vi "UHR-Fleezers Control (host) - 12.7b.vi"() -> ()   [LabVIEW 2012] (continued)
  T23 = typedef "XDNodeRunTimeDep.lvlib/timing_clust.ctl" = cluster{"Expected End [f-1]":u64, "Actual End [f-1]":u64, "Finished Late? [f-1]":bool, "Expected End [i-1]":u64, "Actual End [i-1]":u64, "Finished Late? [i-1]":bool, "Expected Start [i]":u64, "Actual Start [i]":u64, "Expected Start [f]":u64, "Actual Start [f]":u64, "Source Name":string, "Structure Name":string, "Period":i64, "Deadline":i64, "Offset":i64, "Start":i64, "Priority":i32, "Timeout":i32, "Mode":T24, "Wakeup Reason":T25, "Error":errorcluster, "Source Type":string, "Secondary Source Type":string, "Global End Time":u64, "Global Start Time":u64, "Frame Duration":u64, "Iteration Duration":u64, "Assigned CPU":i32, "I/O Scan Engine Mode":u32}
  T24 = typedef "XDNodeRunTimeDep.lvlib/nitl_modes.ctl" = enum32{"No Change", "Process missed periods, maintain original phase", "Discard missed periods, maintain original phase", "Process missed periods, ignore original phase", "Discard missed periods, ignore original phase"}
  T25 = typedef "XDNodeRunTimeDep.lvlib/wakeup.ctl" = enum32{"Normal", "Aborted", "Asynchronous wakeup", "Timing source error", "Timed loop error", "Timeout"}
  T26 = enum32{"Status", "Sample Stage", "Syringe Pump", "Trap Control (RF)", "APD Counting", "Fluorescence Laser Control", "Trap AI", "Video", "FPGA"}
  T27 = enum32{"Status", "Sample Stage", "Syringe Pump", "Trap Control (RF)", "APD Counting", "Fluorescence Laser Control", "Trap AI", "Video", "FPGA", "Misc. Configuration"}
  T28 = enum16{"big-endian, network order", "native, host order", "little-endian"}
  T29 = enum16{"open", "replace", "create", "open or create", "replace or create", "replace or create with confirmation"}
  T30 = cluster{"Scan Range AOD (nm) 2":dbl, "Step Size AOD (nm) 2":dbl, "Scan Speed AOD (nm/s) 2":dbl, "Number of scans (AOD) 2":u16, "Label":string}
  T31 = cluster{"[0]":dbl, "[1]":dbl, "[2]":dbl, "[3]":dbl, "[4]":dbl, "[5]":dbl}
  T32 = cluster{"Diameter (mm)":dbl, "Units":dbl, "Volume":dbl, "Rate":dbl}
  T33 = cluster{"Left":i32, "Top":i32, "Width":u32, "Height":u32}
  T34 = cluster{cluster{"Left":i32, "Top":i32, "Width":u32, "Height":u32}}[]
  T35 = enum32{"Normal Display", "Dual Display (APD)", "FFT", "High Res Display"}
  T36 = cluster{"Origin Pixel":cluster{"X":sgl, "Y":sgl}, "Angle Relative to Horizontal (deg)":sgl, "Axis Reference":u32}
  T37 = typedef "Simple Grid Descriptor" = cluster{"X Step":sgl, "Y Step":sgl, "Unit":T38}
  T38 = typedef "Image Unit" = enum32{"Undefined", "Angström", "Micrometer", "Millimeter", "Centimeter", "Meter", "Kilometer", "Microinch", "Inch", "Feet", "Nautical miles", "Standard miles", "Steps"}
  T39 = cluster{"averaging mode":u16, "weighting mode":u16, "number of averages":u32}
  T40 = cluster{"dB On (F)":bool, "unwrap phase (F)":bool, "convert to degree (F)":bool}
  T41 = cluster{string, string, string, string, string, string, string, string}
  T42 = cluster{string, string, string, string, string, string, string, string, string, string, string, string}
  T43 = cluster{string, string, string, string, string, string, string, string, string, string, string, string, string}
  T44 = cluster{string, string, string, string, string, string, string, string, string, string, string, string, string, string}
  T45 = cluster{"BD 1 Frequency 1 (MHz)":dbl, "BD 1 Frequency 2 (MHz)":dbl}
  T46 = cluster{"f0":dbl, "df":dbl, "magnitude":dbl[]}[][]
  T47 = cluster{"Comment (data description)":string, "Channel 1 Buffer":string, "Channel 2 Buffer":string, "Channel 3 Buffer":string, "Title":string, "DNA Construct":string, "Bead diameter":dbl, "Name":string}
  T48 = enum32{"setting", "request", "request control", "info", "statistics", "system settings", "I/O sub system", "HRT control", "camera descriptions", "device specific data", "event sub system settings", "event sub system results", "image memory manager"}
  T49 = typedef "AviRefnum.ctl" = refnum<k1>
  T50 = typedef "imagedata.ctl" = cluster{"image type":i32, "image depth":i32, "image":u8[], "mask":u8[], "colors":u32[], "Rectangle":cluster{"left":i16, "top":i16, "right":i16, "bottom":i16}}
diagram:
  w13 = u16 10 items=["1.0"=10, "1.5"=15, "2.0"=20] ("stop bits (10: 1 bit)")
  w80 = u16 20 items=["1.0"=10, "1.5"=15, "2.0"=20] ("stop bits (10: 1 bit)")
  w83 = u16 20 items=["1.0"=10, "1.5"=15, "2.0"=20] ("stop bits (10: 1 bit)")
  w109 = u16 20 items=["1.0"=10, "1.5"=15, "2.0"=20] ("stop bits (10: 1 bit)")
  w19 = T18 2 items=["Grayscale (U8)", "Grayscale (I16)", "Grayscale (SGL)", "Complex (CSG)", "RGB (U32)", "HSL (U32)", "RGB (U64)", "Grayscale (U16)"] ("Image Type")
  w239 = 10.0 ("y")
  w238 = 32767.0 ("y")
  w254 = 6.0  # clock mult.
  w255 = 49152000.0  # TCXO frequ.
  # "Trap X limits"
  # "What are these?"
  # "I don't think you need to do this.\nEverytime you want to adjust phase you always set this anyway.\nSince we removed the separate +/- controls.\n\nHaven't added for added fl lasers.  Should remove this code."
  # "Bottom 1 Harvard"
  # "Top 3 Harvard"
  # "Center Harvard"
  # "Bottom 1 Harvard"
  # "Top 3 Harvard"
  # "Center Harvard"
  n1 = Build Array("DIO count 1 (ticks)", "DIO count 2 (ticks)", "DIO count 3 (ticks)") -> (w160:u16[])
  n2 = xnode "Open FPGA VI Reference"("resource name"=T19 "750kHzDAQ") -> ("FPGA VI Reference Out"=w263:T20, "error out"=w262:errorcluster)  [unwired: 1 in]
  n3 = local read "AO1"() -> (w233:dbl)
  n4 = local read "AO2"() -> (w232:dbl)
  n5 = local read "Scan Increment (MHz)"() -> (w250:dbl)
  n6 = local read "Continuous MCL Scanning"() -> (w220:bool)
  n7 = local read "Fast Scan Dir"() -> (w219:bool)
  n8 = xnode "Invoke Method"("FPGA VI Reference In"=w263, "error in"=w262) -> ("FPGA VI Reference Out"=w23:T20, "error out"=w179:errorcluster)
  n9 = local read "Number of scans (MCL)"() -> (w221:u64)
  n10 = Multiply(x=w233, y=w238) -> (x*y=w235:dbl)
  n11 = Multiply(x=w232, y=w238) -> (x*y=w237:dbl)
  n12 = Divide(x=w235, y=w239) -> (x/y=w234:dbl)
  n13 = Divide(x=w237, y=w239) -> (x/y=w236:dbl)
  n14 = To Word Integer(number=w234) -> (16bit integer=w231:i16)
  n15 = To Word Integer(number=w236) -> (16bit integer=w230:i16)
  n16 = Not(x=w219) -> (.not. x?=w214:bool)
  n17 = local read "Cycles/step (MCL)"() -> (w222:u64)
  n18 = Multiply(x=w250, y=1000.0) -> (x*y=w257:dbl)
  n19 = local read "Scan steps (MCL)"() -> (w223:u64)
  n20 = local read "Desired Scan Incr (V)"() -> (w225:dbl)
  n21 = Scale By Power Of 2(n=48, x=w257) -> (x*2^n=w258:dbl)
  n22 = Unbundle By Name(cluster{"output high":i16, "output low":i16} {"output high"=3000, "output low"=0} ("FB output range 1")) -> ("output high"=w61:i16, "output low"=w60:i16)
  n23 = Multiply(x=w255, y=w254) -> (x*y=w253:dbl)
  n24 = Divide(x=w258, y=w253) -> (x/y=w252:dbl)
  n25 = local read "Setpoints (V)"() -> (w269:cluster{"Set 1":dbl, "Set 2":dbl})
  n26 = To Quad Integer(1:w252) -> (0:w249:i64)
  n27 = Divide(x=40000000.0, y="AI Count (ticks)") -> (x/y=w210:dbl)
  n28 = Multiply(x=w225, y=32767.0) -> (x*y=w227:dbl)
  n29 = local read "Trap Intensity PID Gains"() -> (w264:T9)
  n30 = local read "Next trap write delay (ticks)"() -> (w5:u8)
  n31 = local read "XY phase ext loop method"() -> (w4:bool)
  n32 = local read "Amp switch delay 2"() -> (w3:u8)
  n33 = local read "BD 2 Delay (Ticks) 2"() -> (w2:u8)
  n34 = local read "BD 1 Delay (ticks) 2"() -> (w1:u8)
  n35 = local write "Trap Pos FIFO Timeout"(u16 0 ("Trap Pos FIFO Timeout")) -> ()
  n36 = local read "Number Interlace Sets"() -> (w153:u8)
  n37 = Split 1D Array(array=w160, index=w153) -> (first subarray=w162:u16[])  [unwired: 1 out]
  n38 = Add Array Elements(numeric array=w162) -> (sum=w161:u16)
  n39 = local read "# Samples/channel"() -> (w242:u32)
  n40 = local read "Number of F/B Scans (AOD)"() -> (w243:u16)
  n41 = local read "Not-Interlacing Set"() -> (w152:enum32{"Set 1", "Set 2", "Set 3"})
  n42 = To Unsigned Byte Integer(number=w152) -> (unsigned 8bit integer=w158:u8)
  n43 = Index Array(array=w160, index=w158) -> (element=w159:u16)
  n44 = local read "Feedback On/Off"() -> (w272:cluster{"Set 1":bool, "Set 2":bool})
  n45 = local read "BD 2 Delay (Ticks)"() -> (w6:u8)
  n46 = local read "BD 1 Delay (ticks)"() -> (w7:u8)
  n47 = local read "Scan steps (AOD)"() -> (w248:u64)
  n48 = local read "All FB On/Off"() -> (w273:bool)
  n49 = local read "Cycles/step (AOD)"() -> (w247:u64)
  n50 = local write "AI rate (Hz)"(w210) -> ()
  n51 = Divide(x=w227, y=10.0) -> (x/y=w226:dbl)
  n52 = Multiply(x=w248, y=w247) -> (x*y=w246:u64)
  n53 = Unbundle By Name(w264) -> ("proportional gain (Kc)"=w65:i16, "integral gain (Kc*Ts/Ti)"=w64:i16, "derivative gain (Kc*Td/Ts)"=w63:i16)
  n54 = property on="AI Count (ticks)" class="DigNum (strict)"("Val(Sgnl)"="AI Count (ticks)") -> ()  [unwired: 2 in, 2 out]
  n55 = Multiply(x=3276.7, y=w269) -> (x*y=w268:cluster{"Set 1":dbl, "Set 2":dbl})
  n56 = To Word Integer(number=w226) -> (16bit integer=w224:i16)
  n57 = Multiply(x=w246, y=u64 2) -> (x*y=w244:u64)
  n58 = Divide(x=w210, y="FPGA Ave.") -> (x/y=w211:dbl)
  n59 = To Word Integer(number=w268) -> (16bit integer=w267:cluster{"Set 1":i16, "Set 2":i16})
  n60 = Multiply(x=w244, y=w243) -> (x*y=w241:u64)
  n61 = local read "Sets to FIFO (Traps)"() -> (w69:T15)
  n62 = local write "Ave. Rate (Hz)"(w211) -> ()
  n63 = Divide(x=w241, y=w242) -> (x/y=w240:dbl)
  n64 = Unbundle By Name(w267) -> ("Set 1"=w266:i16, "Set 2"=w265:i16)
  n65 = local read "2D or 1D Scan"() -> (w171:bool)
  n66 = local write "Data points/scans"(w241) -> ()
  n67 = local read "Scan BD"() -> (w259:bool)
  n68 = And(x=w272, y=w273) -> (x .and. y?=w271:cluster{"Set 1":bool, "Set 2":bool})
  n69 = local write "Data points/scan (f/b)"(w244) -> ()
  n70 = Reciprocal(x=w211) -> (1/x=w212:dbl)
  n71 = local read "N Acq Sets (Traps + Fl.)"() -> (w203:i16)
  n72 = local write "N sets should be saved"(w240) -> ()
  n73 = Unbundle By Name(w271) -> ("Set 1"=w275:bool, "Set 2"=w274:bool)
  n74 = local read "Interlace"() -> (w154:bool)
  n75 = Select(t=w161, s=w154, f=w159) -> (s? t:f=w151:u16)
  n76 = local write "Update Count (MCL)"(w151) -> ()
  n77 = local write "Total Counts (ticks)"(w151) -> ()
  n78 = local write "Ave. Period (s)"(w212) -> ()
  n79 = Unbundle By Name(w69) -> ("Set 1"=w68:bool, "Set 2"=w67:bool, "Set 3"=w66:bool)
  n80 = property on="2D or 1D Scan" class="Bool (strict)"("Val(Sgnl)"=w171) -> ()  [unwired: 2 in, 2 out]
  n81 = xnode "Read/Write Control"("FPGA VI Reference In"=w170, "error in"=w179, "ai count"="AI Count (ticks)", "Interlace ON/OFF"=w154, "Number Interlace Cycles"=w153, "Set 1"=w68, "Set 2"=w67, "Set 3"=w66, "FB On/Off Set 1"=w275, "FB On/Off Set 2"=w274, "Interlace Off Parameters"=w152, "FB Setpoint Set 1"=w266, "FB Setpoint Set 2"=w265, "P1"=w65, "I1"=w64, "D1"=w63, "FB1 output high"=w61, "FB1 output low"=w60, "Cycles per step"=w247, "Scan BD"=w259, "Number of scans"=w243, "Scan steps"=w248, "Scan freq.  increment"=w249, "AO1"=w231, "AO2"=w230, "Scan freq.  increment (MCL)"=w224, "Scan steps (MCL)"=w223, "Cycles per step (MCL)"=w222, "Number of scans (MCL)"=w221, "MCL count"=w151, "Cont. Scan (MCL)"=w220, "MCL Scan Axis"=w214, "1D or 2D Scan?"=w171, "N of AI1 Int Acq Sets"=w203, "Amp switch delay"="Amp switch delay", "Swap F1 and F2"="Swap F1 and F2", "APD to FIFO"=FALSE, "DIO count 1 (ticks)"="DIO count 1 (ticks)", "DIO count 2 (ticks)"="DIO count 2 (ticks)", "DIO count 3 (ticks)"="DIO count 3 (ticks)", "BD 1 Delay (ticks)"=w7, "BD 2 Delay (Ticks)"=w6, "Next trap write delay (ticks)"=w5, "XY phase ext loop method"=w4, "Amp switch delay 2"=w3, "BD 2 Delay (Ticks) 2"=w2, "BD 1 Delay (ticks) 2"=w1) -> ("FPGA VI Reference Out"=w25:T20, "error out"=w24:errorcluster)  [unwired: 1 in]
  n82 = local read "Laser interlacing mode"() -> (w150:enum32{"Laser ON", "Laser OFF", "Interlace"})
  n83 = local read "Green Laser ON"() -> (w149:bool)
  n84 = local read "Trap Pos. FB Range"() -> (w59:T12)
  n85 = local read "Trap Pos. FB Gains"() -> (w58:T11)
  n86 = Multiply(x="Green Intensity % (FB OFF)", y=655.35) -> (x*y=w142:dbl)
  n87 = local read "Invert laser interlacing"() -> (w38:bool)
  n88 = local read "Trap Pos. AI1 X Pre-scale"() -> (w97:u16)
  n89 = Multiply(x="Green FB Setpoint (mV)", y=3.2767) -> (x*y=w139:dbl)
  n90 = local read "Trap Pos FB Int Count"() -> (w91:u16)
  n91 = local read "Differential FB?"() -> (w85:bool)
  n92 = local read "Neg. TTrig FPGA"() -> (w87:bool)
  n93 = Multiply(x="Red FB Setpoint (mV)", y=3.2767) -> (x*y=w46:dbl)
  n94 = To Unsigned Word Integer(number=w142) -> (unsigned 16bit integer=w140:u16)
  n95 = Multiply(x="Red Intensity % (FB OFF)", y=655.35) -> (x*y=w42:dbl)
  n96 = To Word Integer(number=w139) -> (16bit integer=w137:i16)
  n97 = Unbundle By Name("Green FB Gains") -> ("proportional gain (Kc)"=w50:i16, "integral gain (Kc*Ts/Ti)"=w49:i16, "derivative gain (Kc*Td/Ts)"=w48:i16)
  n98 = Unbundle By Name("Red FB Gains") -> ("proportional gain (Kc)"=w35:i16, "integral gain (Kc*Ts/Ti)"=w34:i16, "derivative gain (Kc*Td/Ts)"=w33:i16)
  n99 = case shown="False" w149 {
    tunnel: w150 -> [_ w301]
    tunnel: [enum32{"Laser ON", "Laser OFF", "Interlace"}."Laser OFF" ("Green laser mode") w301] -> w37
    frame False {
    }
    frame True {
    }
  }
  n100 = To Word Integer(number=w46) -> (16bit integer=w43:i16)
  n101 = Unbundle By Name(w58) -> ("proportional gain (Kc)"=w54:fxp<+/-,16,8>, "integral gain (Kc*Ts/Ti)"=w53:fxp<+/-,16,8>, "derivative gain (Kc*Td/Ts)"=w52:fxp<+/-,16,8>)
  n102 = To Unsigned Word Integer(number=w42) -> (unsigned 16bit integer=w39:u16)
  n103 = Unbundle By Name(w59) -> ("output high"=w57:fxp<+/-,16,1>, "output low"=w55:fxp<+/-,16,1>)
  n104 = local read "Trap Pos FB Monitor\nT1 or T2"() -> (w102:bool)
  n105 = local read "Trap Pos FB Negate Action"() -> (w101:bool)
  n106 = local read "Trap Pos. FB Offset Factor"() -> (w100:i64)
  n107 = local read "Trap Pos. FB Mult Factor"() -> (w99:i64)
  n108 = xnode "Read/Write Control"("FPGA VI Reference In"=w25, "error in"=w24, "Invert GI 2"=w38, "Operating Mode 2"=w37, "P3"=w50, "I3"=w49, "D3"=w48, "Green FB Setpoint"=w137, "Green FB On/Off"="Green FB On/Off", "Current Out"=w140, "Green int current ON count adj"="Green int current ON count adj", "Operating Mode"=w37, "Invert GI"=w38, "Trap Pos FB Monitor T1 or T2"=w102, "Trap Pos FB Negate Action"=w101, "Trap Pos. FB Offset Factor"=w100, "Trap Pos. FB Mult Factor"=w99, "Force feedback"=FALSE, "AI1 X Scale"=w97, "Trap Pos to FIFO"=TRUE, "Trap Pos FB Int Count"=w91, "TTrig Negate Pos"=w87, "FB Trig Integrate"="FB Trig Integrate", "Diff FB Measurement?"=w85, "Negate Diff?"="Negate Diff?", "P2"=w54, "I2"=w53, "D2"=w52, "FB2 output high"=w57, "FB2 output low"=w55, "Red FB Setpoint"=w43, "RI Current Out"=w39, "Red Laser Operating Mode"=w37, "RI Operating Mode 2"=w37, "Invert RI 2"=w38, "Invert RI"=w38, "P4"=w35, "I4"=w34, "D4"=w33, "Red FB On/Off"="Red FB On/Off") -> ("FPGA VI Reference Out"=w29:T20, "error out"=w31:errorcluster)
  n109 = stacked-sequence {
    tunnel: w31 -> [_ _ _ w312]
    tunnel: [_ _ _ w312] -> w30
    tunnel: w29 -> [_ _ _ w313]
    tunnel: [_ _ _ w313] -> w28
    frame #0 {
      w302 = T21."empty" ("mode")
      # "Clear external fluorescence triggering FIFO"
      # "APD loop counts"
      # "Fluorescence loop counts (rates)"
      n110 = local read "APD Integration Time (s)"() -> (w304:dbl)
      n111 = local read "Interlace ON count"() -> (w305:u16)
      n112 = call "Smart Buffer (DBL) 1.vi"("mode"=w302) -> ()  [unwired: 5 in, 6 out]
      n113 = call "Smart Buffer (DBL) 2.vi"("mode"=w302) -> ()  [unwired: 5 in, 6 out]
      n114 = property on="APD Integration Time (s)" class="DigNum (strict)"("Val(Sgnl)"=w304) -> ()  [unwired: 2 in, 2 out]
      n115 = property on="Interlace ON count" class="DigNum (strict)"("Val(Sgnl)"=w305) -> ()  [unwired: 2 in, 2 out]
      "Number of APDs" <- 3.0 ("Number of APDs")
    }
    frame #1 {
      # "Number of APDs affects\nAPD DMA transfer"
      # "General settings for all lasers:"
      # "And includes all laser\nON/OFF settings"
      # "Fluorescent lasers settings:"
      # "Blue laser settings:"
      n116 = local read "Laser interlacing mode"() -> (w307:enum32{"Laser ON", "Laser OFF", "Interlace"})
      n117 = local read "Invert laser interlacing"() -> (w306:bool)
      n118 = local read "Blue FB On/Off"() -> (w308:bool)
      n119 = property on="Blue FB On/Off" class="Bool (strict)"("Val(Sgnl)"=w308) -> ()  [unwired: 2 in, 2 out]
      n120 = property on="Invert laser interlacing" class="Bool (strict)"("Val(Sgnl)"=w306) -> ()  [unwired: 2 in, 2 out]
      n121 = property on="Laser interlacing mode" class="RadioBtnsControl (strict)"("Val(Sgnl)"=w307) -> ()  [unwired: 2 in, 2 out]
    }
    frame #2 {
      w309 = path "C:/Home/wheeler/Comstock-LabView-Link.udl" ("connection information")
      # "Initialize the database connection"
      n122 = call-poly <vilib>:"DB Tools Open Connection.vi"("connection information"=w309) -> ("connection reference"=w310:T17)  [unwired: 7 in, 1 out]
      "connection reference" <- w310
      n123 = local write "connection reference"(w310) -> ()
      n124 = local write "Database link"(w309) -> ()
    }
    frame #3 {
      n125 = Wait (ms)(milliseconds to wait=u32 1000) -> ()  [unwired: 1 out]
    }
  }
  n126 = local write "Offset (nm)"(0.0 ("Offset (nm)")) -> ()
  n127 = local write "Bead Mean (nm)"(0.0 ("Bead Mean (nm)")) -> ()
  n128 = case shown="\"2axisAOD\"" "1axis AOM vs 2 axis AOD" {
    tunnel: [T16 {"Minimum"=0.0, "Maximum"=40.0, "Increment"=0.1} ("Min Max Inc") T16 {"Minimum"=60.0, "Maximum"=90.0, "Increment"=1.0} ("Min Max Inc")] -> w10
    tunnel: [T16 {"Minimum"=0.0, "Maximum"=45.0, "Increment"=1.0} ("Data Entry Limits") T16 {"Minimum"=0.0, "Maximum"=50.0, "Increment"=1.0} ("Data Entry Limits")] -> w8
    frame "2axisAOD" {
      w315 = 35.0 ("BD 1 Amplitude 1 (%)")
      w316 = 30.0 ("BD 1 Frequency 1 (MHz)")
      # "Amp Limits"
      # "Freq Limits"
      n129 = local write "BD 2 Delay (Ticks)"(u8 47 ("BD 2 Delay (Ticks)")) -> ()
      n130 = local write "All FB On/Off"(FALSE ("All FB On/Off")) -> ()
      n131 = local write "Number Interlace Sets"(u8 2 ("Number Interlace Sets")) -> ()
      n132 = local write "BD 1 Frequency 1 (MHz)"(w316) -> ()
      n133 = local write "BD 1 Frequency 2 (MHz)"(w316) -> ()
      n134 = local write "BD 1 Amplitude 2 (%)"(w315) -> ()
      n135 = local write "BD 1 Amplitude 1 (%)"(w315) -> ()
      n136 = local write "BD 2 Frequency 1 (MHz)"(w316) -> ()
      n137 = local write "BD 2 Amplitude 1 (%)"(w315) -> ()
      n138 = local write "BD 2 Frequency 2 (MHz)"(w316) -> ()
      n139 = local write "BD 2 Amplitude 2 (%)"(w315) -> ()
    }
    frame "1axis", Default {
      # "Amp Lmits"
      # "Freq Limits"
    }
  }
  n140 = xnode "Invoke Method"("FPGA VI Reference In"=w28, "error in"=w30, "Requested Depth"="Trap AI FIFO Depth") -> ("FPGA VI Reference Out"=w105:T20, "error out"=w104:errorcluster)  [unwired: 1 out]
  n141 = xnode "Invoke Method"("FPGA VI Reference In"=w105, "error in"=w104, "Requested Depth"="Trap Position FIFO Depth") -> ("FPGA VI Reference Out"=w93:T20, "error out"=w92:errorcluster)  [unwired: 1 out]
  n142 = flat-sequence "Safety limits on RF frequencies and amplitudes (for AOM protection)" {
    tunnel: w23 -> [w327]
    tunnel: [w327] -> w170
    tunnel: [w324] -> w169
    tunnel: [w323] -> w168
    tunnel: [w325] -> w166
    tunnel: [w326] -> w167
    tunnel: w10 -> [w324]
    tunnel: w8 -> [w323]
    frame #0 {
      w326 = T16 {"Minimum"=0.0, "Maximum"=40.0, "Increment"=0.1} ("Min Max Inc")
      w325 = T16 {"Minimum"=0.0, "Maximum"=45.0, "Increment"=1.0} ("Data Entry Limits")
      n143 = property on="BD 2 Frequency 1 (MHz)" class="DigNum (strict)"("Data Range"=w326) -> ()  [unwired: 2 in, 2 out]
      n144 = property on="BD 2 Frequency 3 (MHz)" class="DigNum (strict)"("Data Range"=w326) -> ()  [unwired: 2 in, 2 out]
      n145 = property on="BD 2 Frequency 2 (MHz)" class="DigNum (strict)"("Data Range"=w326) -> ()  [unwired: 2 in, 2 out]
      n146 = property on="BD 1 Frequency 1 (MHz)" class="DigNum (strict)"("Data Range"=w324) -> ()  [unwired: 2 in, 2 out]
      n147 = property on="BD 1 Frequency 2 (MHz)" class="DigNum (strict)"("Data Range"=w324) -> ()  [unwired: 2 in, 2 out]
      n148 = property on="BD 1 Frequency 3 (MHz)" class="DigNum (strict)"("Data Range"=w324) -> ()  [unwired: 2 in, 2 out]
      n149 = property on="BD 2 Amplitude 1 (%)" class="DigNum (strict)"("Data Range"=w325) -> ()  [unwired: 2 in, 2 out]
      n150 = property on="BD 2 Amplitude 2 (%)" class="DigNum (strict)"("Data Range"=w325) -> ()  [unwired: 2 in, 2 out]
      n151 = property on="BD 2 Amplitude 3 (%)" class="DigNum (strict)"("Data Range"=w325) -> ()  [unwired: 2 in, 2 out]
      n152 = property on="BD 1 Amplitude 3 (%)" class="DigNum (strict)"("Data Range"=w323) -> ()  [unwired: 2 in, 2 out]
      n153 = property on="BD 1 Amplitude 2 (%)" class="DigNum (strict)"("Data Range"=w323) -> ()  [unwired: 2 in, 2 out]
      n154 = property on="BD 1 Amplitude 1 (%)" class="DigNum (strict)"("Data Range"=w323) -> ()  [unwired: 2 in, 2 out]
      "X RF Frequency Limits (MHz)" <- w324
      "X RF Amplitude Limits (%)" <- w323
      "Y RF Amplitude Limits (%)" <- w325
      "Y RF Frequency Limits (MHz)" <- w326
    }
  }
  n155 = xnode "Invoke Method"("FPGA VI Reference In"=w93, "error in"=w92) -> ("FPGA VI Reference Out"=w178:T20, "error out"=w177:errorcluster)  [unwired: 1 in]
  n156 = flat-sequence "Initial FPGA Loop Relative Phase Adjustment" {
    tunnel: "Initial Phase Adjustment (AI1)" -> [w342]
    tunnel: "Initial Phase Adjustment (GI)" -> [w341]
    tunnel: w178 -> [w340]
    tunnel: w177 -> [w339]
    tunnel: "Initial Phase Adj. (MCL)" -> [w338]
    tunnel: [w343] -> w187
    tunnel: [w337] -> w183
    tunnel: "Initial Phase Adjustment (APD Acq)" -> [w336]
    tunnel: "Initial Phase Adjustment (APD 1 Gate)" -> [w335]
    tunnel: "Initial Phase Adjustment (Green FB)" -> [w334]
    tunnel: "Initial Phase Adjustment (GI) 2" -> [w333]
    tunnel: "Initial Phase Adjustment (APD 2 Gate)" -> [w332]
    tunnel: "Initial Phase Adjustment (RI)" -> [w331]
    tunnel: "Initial Phase Adjustment (BI DO)" -> [w330]
    tunnel: "Initial Phase Adjustment (BI AO)" -> [w329]
    tunnel: "Initial Phase Adjustment (APD 3 Gate)" -> [w328]
    tunnel: w187 -> [w345]
    tunnel: [w346] -> w184
    tunnel: w183 -> [w346]
    tunnel: [w345] -> w182
    tunnel: w184 -> [w349]
    tunnel: w182 -> [w348]
    tunnel: [w351] -> w181
    tunnel: [w350] -> w180
    tunnel: [w353] -> w185
    tunnel: [w354] -> w186
    tunnel: w181 -> [w354]
    tunnel: w180 -> [w353]
    frame #0 {
      n157 = xnode "Read/Write Control"("FPGA VI Reference In"=w340, "error in"=w339, "Phase count adjustment"=w342, "Phase count adjustment (GI)"=w341, "Phase count adjustment (MCL)"=w338, "Phase Count Adjustment (APD Acq)"=w336, "Phase count adjustment (APD 1 Gate)"=w335, "Phase count adjustment (APD 2 Gate)"=w332, "Phase count adjustment (Green FB)"=w334, "Phase count adjustment (GI) 2"=w333, "Phase count adjustment (RI)"=w331, "Phase count adjustment (BI AO)"=w329, "Phase count adjustment (BI D)"=w330, "Phase count adjustment (APD 3 Gate)"=w328) -> ("FPGA VI Reference Out"=w337:T20, "error out"=w343:errorcluster)
    }
    frame #1 {
      n158 = Wait (ms)(milliseconds to wait=u32 100) -> ()  [unwired: 1 out]
    }
    frame #2 {
      w347 = TRUE
      n159 = xnode "Read/Write Control"("FPGA VI Reference In"=w349, "error in"=w348, "+ phase"=w347, "+ phase (GI)"=w347, "+ phase (MCL)"=w347, "+ phase (APD Acq)"=w347, "+ phase (APD 1 Gate)"=w347, "+ phase (APD 2 Gate)"=w347, "+ phase (Green FB)"=w347, "+ phase (GI) 2"=w347, "+ phase (RI)"=w347, "+ phase (BI AO)"=w347, "+ phase (BI D)"=w347, "+ phase (APD 3 Gate)"=w347) -> ("FPGA VI Reference Out"=w350:T20, "error out"=w351:errorcluster)
    }
    frame #3 {
      n160 = Wait (ms)(milliseconds to wait=u32 100) -> ()  [unwired: 1 out]
    }
  }
  n161 = local read "Phase adj. (Green FB)"() -> (w163:i16)
  n162 = local read "Phase adj. (GI) 2"() -> (w143:i16)
  n163 = local read "Phase adjust (MCL)"() -> (w215:i16)
  n164 = local read "Phase adj. (AI1)"() -> (w217:i16)
  n165 = local read "Phase adj. (GI)"() -> (w216:i16)
  n166 = xnode "Read/Write Control"("FPGA VI Reference In"=w185, "error in"=w186, "Phase count adjustment"=w217, "Phase count adjustment (GI)"=w216, "Phase count adjustment (MCL)"=w215, "Phase Count Adjustment (APD Acq)"="Phase Adj. (APD Acq)", "Phase count adjustment (APD 1 Gate)"="Phase Adj. (APD 1 Gate)", "Phase count adjustment (APD 2 Gate)"="Phase Adj. (APD 2 Gate)", "Phase count adjustment (Green FB)"=w163, "Phase count adjustment (GI) 2"=w143) -> ("FPGA VI Reference Out"=w129:T20, "error out"=w192:errorcluster)
  n167 = call "Initialize RF boards - interlace 3.vi"("error in"=w192, "FPGA VI Reference In"=w129) -> ("error out"=w190:errorcluster, "FPGA VI Reference Out"=w191:T20)
  n168 = call "set RF board frequency - interlace.vi"("Board 2 Frequency Limits"=w167, "Board 1 Frequency Limits"=w169, "error in"=w190, "FPGA VI Reference In"=w191, "Board 2 Frequency 3 (MHz)"="BD 2 Frequency 3 (MHz)", "Board 1 Frequency 3 (MHz)"="BD 1 Frequency 3 (MHz)", "Board 2 Frequency 2 (MHz)"="BD 2 Frequency 2 (MHz)", "Board 2 Frequency 1 (MHz)"="BD 2 Frequency 1 (MHz)", "Board 1 Frequency 2 (MHz)"="BD 1 Frequency 2 (MHz)", "Board 1 Frequency 1  (MHz)"="BD 1 Frequency 1 (MHz)") -> ("error out"=w290:errorcluster, "FPGA VI Reference Out"=w291:T20)
  n169 = call "set RF board amplitude - interlace.vi"("Board 2 Amplitude Limits"=w166, "Board 1 Amplitude Limits"=w168, "error in"=w290, "FPGA VI Reference In"=w291, "Board 2 Amplitude 3 (%)"="BD 2 Amplitude 3 (%)", "Board 1 Amplitude 3 (%)"="BD 1 Amplitude 3 (%)", "Board 2 Amplitude 2 (%)"="BD 2 Amplitude 2 (%)", "Board 2 Amplitude 1 (%)"="BD 2 Amplitude 1 (%)", "Board 1 Amplitude 2 (%)"="BD 1 Amplitude 2 (%)", "Board 1 Amplitude 1 (%)"="BD 1 Amplitude 1 (%)") -> ("error out"=w278:errorcluster, "FPGA VI Reference Out"=w279:T20)
  n170 = flat-sequence {
    tunnel: w279 -> [w364]
    tunnel: w278 -> [w363]
    tunnel: [w362] -> w283
    tunnel: [w361] -> w282
    tunnel: [w368] -> w281
    tunnel: w283 -> [w368]
    tunnel: [w367] -> w280
    tunnel: w282 -> [w367]
    tunnel: w281 -> [w377]
    tunnel: w280 -> [w376]
    tunnel: [w375] -> w22
    tunnel: [w374] -> w94
    frame #0 {
      w355 = FALSE ("Retract Pump 3")
      n171 = local read "Trap 1 (ON/OFF)"() -> (w356:bool)
      n172 = xnode "Read/Write Control"("FPGA VI Reference In"=w364, "error in"=w363, "Direct RF Box  Communication"=FALSE) -> ("FPGA VI Reference Out"=w362:T20, "error out"=w361:errorcluster)
      n173 = local write "Saving..."(FALSE ("Saving Data")) -> ()
      n174 = local write "Stop All"(FALSE ("Stop All")) -> ()
      n175 = local write "Retract Pump 1"(w355) -> ()
      n176 = local write "Retract Pump 3"(w355) -> ()
      n177 = local write "Index"(1.0 ("Index")) -> ()
      n178 = property on="Trap 1 ON" class="Bool (strict)"("Value"=w356) -> ()  [unwired: 2 in, 2 out]
      "Manipulating Trap" <- FALSE ("Manipulating Trap")
    }
    frame #1 {
      n179 = local read "Trap 2 (ON/OFF)"() -> (w366:bool)
      n180 = Wait (ms)(milliseconds to wait=u32 10) -> ()  [unwired: 1 out]
      n181 = property on="Trap 2 ON" class="Bool (strict)"("Val(Sgnl)"=w366) -> ()  [unwired: 2 in, 2 out]
    }
    frame #2 {
      n182 = local read "Scan Range (nm)"() -> (w370:dbl)
      n183 = xnode "Read/Write Control"("FPGA VI Reference In"=w377, "error in"=w376, "FPGA Controls  RF Box"=TRUE ("Direct RF Box  Communication")) -> ("FPGA VI Reference Out"=w375:T20, "error out"=w374:errorcluster)
      n184 = call "Update messages.vi"("Message to add"="UHR-Fleezers ready.", "Old message string"="") -> ("New message string"=w373:string)
      n185 = local write "Messages"(w373) -> ()
      n186 = property on="Scan Range (nm)" class="DigNum (strict)"("Val(Sgnl)"=w370) -> ()  [unwired: 2 in, 2 out]
    }
  }
  n187 = Subtract(x="BD 1 Frequency 1 (MHz)", y="BD 1 Frequency 2 (MHz)") -> (x-y=w202:dbl)
  n188 = Subtract(x="BD 2 Frequency 1 (MHz)", y="BD 2 Frequency 2 (MHz)") -> (x-y=w201:dbl)
  n189 = Square(x=w201) -> (x^2=w199:dbl)
  n190 = Square(x=w202) -> (x^2=w200:dbl)
  n191 = Add(x=w200, y=w199) -> (x+y=w198:dbl)
  n192 = Square Root(x=w198) -> (sqrt(x)=w197:dbl)
  n193 = local write "Trap Delta (MHz)"(w197) -> ()
  n194 = call-poly "VISA Configure Serial Port"("VISA resource name"="VISA resource name", "baud rate (9600)"=u32 115200, "stop bits (10: 1 bit)"=w13) -> ("VISA resource name out"=w12:refnum<visa-resource-name>, "error out"=w11:errorcluster)  [unwired: 4 in, 7 out]
  n195 = call-poly "VISA Configure Serial Port"("VISA resource name"="Bottom  1 Harvard Syringe Pump Serial Port", "baud rate (9600)"=u32 115200, "stop bits (10: 1 bit)"=w80) -> ("VISA resource name out"=w76:refnum<visa-resource-name>, "error out"=w75:errorcluster)  [unwired: 4 in, 7 out]
  n196 = call-poly "VISA Configure Serial Port"("VISA resource name"="Top 3 Harvard Syringe Pump Serial Port", "baud rate (9600)"=u32 115200, "stop bits (10: 1 bit)"=w83) -> ("VISA resource name out"=w78:refnum<visa-resource-name>, "error out"=w77:errorcluster)  [unwired: 4 in, 7 out]
  n197 = call-poly "VISA Configure Serial Port"("VISA resource name"="Sample Chamber Stage Serial Port") -> ("VISA resource name out"=w124:refnum<visa-resource-name>, "error out"=w125:errorcluster)  [unwired: 5 in, 8 out]
  "Stage Control Serial Error" <- w125
  n198 = local write "Blue Error Out"(w11) -> ()
  n199 = call-poly "VISA Configure Serial Port"("VISA resource name"="Center Harvard Syringe Pump Serial Port", "baud rate (9600)"=u32 115200, "stop bits (10: 1 bit)"=w109) -> ("VISA resource name out"=w106:refnum<visa-resource-name>, "error out"=w107:errorcluster)  [unwired: 4 in, 7 out]
  n200 = call "IMAQ Create"("Image Name"="APD 1 Image", "Image Type"=w19) -> ("New Image"=w115:T2)  [unwired: 3 in, 1 out]
  n201 = call "IMAQ Create"("Image Name"="APD 2 Image", "Image Type"=w19) -> ("New Image"=w114:T2)  [unwired: 3 in, 1 out]
  n202 = call "IMAQ Create"("Image Name"="APD 3 Image", "Image Type"=w19) -> ("New Image"=w18:T2)  [unwired: 3 in, 1 out]
  n203 = call "IMAQ Create"("Image Name"="Det. X Image", "Image Type"=w19) -> ("New Image"=w113:T2)  [unwired: 3 in, 1 out]
  n204 = call "IMAQ Create"("Image Name"="Det. Y Image", "Image Type"=w19) -> ("New Image"=w112:T2)  [unwired: 3 in, 1 out]
  n205 = Bundle("New Image"=w115, "New Image"=w114, "New Image"=w18, "New Image"=w113, "New Image"=w112) -> (w111:T22)  [unwired: 1 in]
  n206 = node-c288() -> (w120:T23)  [unwired: 4 in]
  n207 = timed-loop "Run Scripts, including: stage motion" {
    tunnel: w125 -> [w386]
    tunnel: w124 -> [w387]
    tunnel: [w387] -> w123
    tunnel: [w386] -> w122
    timing: w120 -> [_]
    timing-out: [_] -> w119
    tunnel: w106 -> [w385]
    tunnel: w107 -> [w384]
    tunnel: w78 -> [w381]
    tunnel: w77 -> [w380]
    tunnel: w76 -> [w382]
    tunnel: w75 -> [w383]
    tunnel: w12 -> [w379]
    stop <- w388 stop-if-true
    n208 = node-c288() -> ()  [unwired: 1 in, 1 out]
    n209 = event shown="[22] \"Move in a Circle\": Value Change" {
      selector: _ -> [_ _ _ _ _ _ _ _ _ _ _ _ _ _ _ _ _ _ _ _ _ _ _ _]
      dyn-events: _ -> [_ _ _ _ _ _ _ _ _ _ _ _ _ _ _ _ _ _ _ _ _ _ _ _]
      timeout: _ -> [_ _ _ _ _ _ _ _ _ _ _ _ _ _ _ _ _ _ _ _ _ _ _ _]
      tunnel: ["Set Position" "Move to Position" _ _ _ _ _ _ "Read Harvard" _ _ _ _ _ _ "Got ADig bead" "Force FB Data\nScript" _ "Got DNA bead" "Take Stepping Data" _ "Take Detection Laser\nImage" _ _] -> _
      tunnel: [_ _ _ _ _ _ _ _ _ _ _ _ _ _ _ _ _ _ _ _ _ _ _ w1142] -> w388
      tunnel: w386 -> [w406 w414 w427 w457 _ _ _ _ _ w573 w613 w694 w723 w855 w881 _ w917 _ _ _ _ _ _ _]
      tunnel: w387 -> [w407 w415 w428 w458 _ _ _ _ _ w574 w614 w695 w724 w856 w882 _ w918 _ _ _ _ _ _ _]
      tunnel: w385 -> [_ _ _ _ _ _ _ _ w558 _ _ _ _ _ _ _ _ _ _ _ _ _ _ _]
      tunnel: w384 -> [_ _ _ _ _ _ _ _ w557 _ _ _ _ _ _ _ _ _ _ _ _ _ _ _]
      tunnel: w383 -> [_ _ _ _ _ _ _ _ _ _ _ _ _ _ _ _ _ _ _ _ _ _ _ _]
      tunnel: w382 -> [_ _ _ _ _ _ _ _ _ _ _ _ _ _ _ _ _ _ _ _ _ _ _ _]
      tunnel: w381 -> [_ _ _ _ _ _ _ _ _ _ _ _ _ _ _ _ _ _ _ _ _ _ _ _]
      tunnel: w380 -> [_ _ _ _ _ _ _ _ _ _ _ _ _ _ _ _ _ _ _ _ _ _ _ _]
      tunnel: w379 -> [_ _ _ _ w485 w513 w537 w548 _ _ _ _ _ _ _ _ _ _ _ _ _ _ _ w1141]
      event "Set Position", "Set Position 2", "Set Position 3", "Set Position 4", "Set Position 5", "Set Position 1": Value Change {
        n210 = event-data() -> ()  [unwired: 1 in, 5 out]
        n211 = Build Array("Set Position 1", "Set Position 2", "Set Position 3", "Set Position 4", "Set Position 5") -> (w405:bool[])
        n212 = Boolean Array To Number(Boolean array=w405) -> (number=w404:u32)
        n213 = Logarithm Base 2(1:w404) -> (0:w396:dbl)
        n214 = call "Read Stage Position.vi"("error in"=w406, "VISA resource name in"=w407) -> ("Current Position"=w411:cluster{dbl, dbl, dbl}, "error out"=w410:errorcluster)  [unwired: 2 out]
        n215 = Decrement(x="Position") -> (x-1=w394:dbl)
        n216 = Greater Or Equal?(x=w396, y=0.0) -> (x >= y?=w397:bool)
        n217 = Cluster To Array(cluster=w411) -> (array=w408:dbl[])
        n218 = local write "Stage Control Serial Error"(w410) -> ()
        n219 = Select(t=w396, s=w397, f=w394) -> (s? t:f=w393:dbl)
        n220 = Increment(x=w393) -> (x+1=w392:dbl)
        n221 = Build Array (concatenate)(w392, w408) -> (w391:dbl[])
        n222 = Replace Array Subset(array="Saved Stage Positions", new element=w391, index (row)=w393) -> (w409:dbl[][])  [unwired: 1 in]
        n223 = local write "Saved Stage Positions"(w409) -> ()
      }
      event "Move to Position": Value Change {
        n224 = event-data() -> ()  [unwired: 1 in, 5 out]
        n225 = flat-sequence {
          tunnel: w415 -> [w419]
          tunnel: w414 -> [w418]
          frame #0 {
            n226 = local read "Saved Stage Positions"() -> (w421:dbl[][])
            n227 = local read "Position"() -> (w420:dbl)
            n228 = local write "Stage Moving"(TRUE ("Stage Moving")) -> ()
            n229 = call "move to saved stage position.vi"("error in"=w418, "Stage VISA resource name in"=w419, "Position"=w420, "Saved Stage Positions"=w421) -> ("error out"=w417:errorcluster)  [unwired: 1 out]
            n230 = local write "Stage Control Serial Error"(w417) -> ()
          }
          frame #1 {
            n231 = call <vilib>:"Beep.vi"() -> ()  [unwired: 3 in, 9 out]
            n232 = local write "Stage Moving"(FALSE ("Stage Moving")) -> ()
          }
        }
      }
      event "Move Cap. 1 (DNA Bottom)": Value Change {
        n233 = event-data() -> ()  [unwired: 1 in, 5 out]
        n234 = local write "Move Cap. 1 (DNA Bottom)"(FALSE ("Move Cap. 1 (DNA Right)")) -> ()
        n235 = flat-sequence {
          tunnel: w427 -> [w430]
          tunnel: w428 -> [w431]
          tunnel: [w431] -> w425
          tunnel: [w430] -> w424
          tunnel: w425 -> [w433]
          tunnel: w424 -> [w432]
          frame #0 {
            n236 = property on="Sample Channel\nFlow" class="Bool (strict)"("Val(Sgnl)"="Cap 1 Samp Flow ON") -> ()  [unwired: 2 in, 2 out]
          }
          frame #1 {
            n237 = local read "Saved Stage Positions"() -> (w443:dbl[][])
            n238 = local write "Stage Moving"(TRUE ("Stage Moving")) -> ()
            n239 = Array Subset(array=w443, index (row)=0 ("index"), length (row)=1 ("length"), index (col)=1 ("index"), length (col)=3 ("length")) -> (w440:dbl[][])
            n240 = Reshape Array(w440, 3 ("dimension size")) -> (w438:dbl[])
            n241 = Array To Cluster(array=w438) -> (cluster=w437:cluster{"[0]":dbl, "[1]":dbl, "[2]":dbl})
            n242 = call "Set Stage Position.vi"("Position"=w437, "error in"=w432, "VISA resource name in"=w433) -> ("error out"=w436:errorcluster)  [unwired: 2 out]
            n243 = local write "Stage Control Serial Error"(w436) -> ()
          }
          frame #2 {
            n244 = local write "Stage Moving"(FALSE ("Stage Moving")) -> ()
            n245 = case shown="True" "Cap 1 Flow ON" {
              frame False {
              }
              frame True {
                n246 = property on="Inject Pump 1" class="Bool (strict)"("Val(Sgnl)"=TRUE ("Value (Signaling)")) -> ()  [unwired: 2 in, 2 out]
              }
            }
            n247 = call <vilib>:"Beep.vi"() -> ()  [unwired: 3 in, 9 out]
          }
          frame #3 {
            n248 = property on="Sample Channel\nFlow" class="Bool (strict)"("Val(Sgnl)"=FALSE ("Value (Signaling)")) -> ()  [unwired: 2 in, 2 out]
            n249 = local read "Cap. 2 BD T1?\n(ADig T1, DNA T2)"() -> (w450:bool)
            n250 = case shown="True" w450 {
              tunnel: "Cap 1 T ON" -> [w452 w453]
              frame False {
                n251 = property on="Trap 1 (ON/OFF)" class="Bool (strict)"("Val(Sgnl)"=w452) -> ()  [unwired: 2 in, 2 out]
              }
              frame True {
                n252 = property on="Trap 2 (ON/OFF)" class="Bool (strict)"("Val(Sgnl)"=w453) -> ()  [unwired: 2 in, 2 out]
              }
            }
            n253 = property on="Got DNA bead" class="Bool"("Key Focus"=TRUE) -> ()  [unwired: 2 in, 2 out]
          }
        }
      }
      event "Move Cap. 2 (ADig Top)": Value Change {
        n254 = event-data() -> ()  [unwired: 1 in, 5 out]
        n255 = local write "Move Cap. 2 (ADig Top)"(FALSE ("Move Cap. 2 (ADig Left)")) -> ()
        n256 = flat-sequence {
          tunnel: w457 -> [w460]
          tunnel: w458 -> [w461]
          tunnel: [w461] -> w455
          tunnel: [w460] -> w454
          tunnel: w455 -> [w464]
          tunnel: w454 -> [w463]
          frame #0 {
            n257 = property on="Sample Channel\nFlow" class="Bool (strict)"("Val(Sgnl)"="Cap 2 Samp Flow ON") -> ()  [unwired: 2 in, 2 out]
          }
          frame #1 {
            w462 = FALSE ("Value (Signaling)")
            n258 = local read "Saved Stage Positions"() -> (w474:dbl[][])
            n259 = local write "Stage Moving"(TRUE ("Stage Moving")) -> ()
            n260 = Array Subset(array=w474, index (row)=1 ("index"), length (row)=1 ("length"), index (col)=1 ("index"), length (col)=3 ("length")) -> (w471:dbl[][])
            n261 = Reshape Array(w471, 3 ("dimension size")) -> (w469:dbl[])
            n262 = property on="Trap 1 (ON/OFF)" class="Bool (strict)"("Val(Sgnl)"=w462) -> ()  [unwired: 2 in, 2 out]
            n263 = property on="Trap 1 (ON/OFF)" class="Bool (strict)"("Val(Sgnl)"=w462) -> ()  [unwired: 2 in, 2 out]
            n264 = Array To Cluster(array=w469) -> (cluster=w468:cluster{"[0]":dbl, "[1]":dbl, "[2]":dbl})
            n265 = call "Set Stage Position.vi"("Position"=w468, "error in"=w463, "VISA resource name in"=w464) -> ("error out"=w467:errorcluster)  [unwired: 2 out]
            n266 = local write "Stage Control Serial Error"(w467) -> ()
          }
          frame #2 {
            n267 = local write "Stage Moving"(FALSE ("Stage Moving")) -> ()
            n268 = call <vilib>:"Beep.vi"() -> ()  [unwired: 3 in, 9 out]
            n269 = case shown="True" "Cap 2 Flow ON" {
              frame False {
              }
              frame True {
                n270 = property on="Inject Pump 3" class="Bool (strict)"("Val(Sgnl)"=TRUE ("Value (Signaling)")) -> ()  [unwired: 2 in, 2 out]
              }
            }
          }
          frame #3 {
            n271 = property on="Sample Channel\nFlow" class="Bool (strict)"("Val(Sgnl)"=FALSE ("Value (Signaling)")) -> ()  [unwired: 2 in, 2 out]
            n272 = case shown="False" "Cap. 2 BD T1?\n(ADig T1, DNA T2)" {
              tunnel: "Cap 2 T ON" -> [w483 w484]
              frame False {
                n273 = property on="Trap 2 (ON/OFF)" class="Bool (strict)"("Val(Sgnl)"=w483) -> ()  [unwired: 2 in, 2 out]
              }
              frame True {
                n274 = property on="Trap 1 (ON/OFF)" class="Bool (strict)"("Val(Sgnl)"=w484) -> ()  [unwired: 2 in, 2 out]
              }
            }
            n275 = property on="Got ADig bead" class="Bool"("Key Focus"=TRUE) -> ()  [unwired: 2 in, 2 out]
          }
        }
      }
      event "Initialize Blue Laser": Value Change {
        n276 = event-data() -> ()  [unwired: 1 in, 5 out]
        n277 = flat-sequence {
          tunnel: w485 -> [w504]
          frame #0 {
            n278 = Concatenate Strings("slmp ", "Blue Laser\nModulation\nPower (mW)") -> (w503:string)
            n279 = call "serial write macro.vi"("String"=w503, "Delay (ms)"="Delay (ms)", "VISA resource name"=w504) -> ("read buffer"=w492:string, "error out"=w493:errorcluster, "VISA resource name out"=w500:refnum<visa-resource-name>)
            n280 = local write "read blue buffer"(w492) -> ()
            n281 = local write "Blue Error Out"(w493) -> ()
            n282 = call "serial write macro.vi"("String"="sdmes 1", "Delay (ms)"="Delay (ms)", "VISA resource name"=w500) -> ("read buffer"=w490:string, "error out"=w491:errorcluster, "VISA resource name out"=w498:refnum<visa-resource-name>)
            n283 = local write "Blue Error Out"(w491) -> ()
            n284 = local write "read blue buffer"(w490) -> ()
            n285 = call "serial write macro.vi"("String"="sames 1", "Delay (ms)"="Delay (ms)", "VISA resource name"=w498) -> ("read buffer"=w487:string, "error out"=w489:errorcluster, "VISA resource name out"=w495:refnum<visa-resource-name>)
            n286 = local write "read blue buffer"(w487) -> ()
            n287 = local write "Blue Error Out"(w489) -> ()
            n288 = call "serial write macro.vi"("String"="l1", "Delay (ms)"="Delay (ms)", "VISA resource name"=w495) -> ("read buffer"=w486:string, "error out"=w488:errorcluster)  [unwired: 1 out]
            n289 = local write "read blue buffer"(w486) -> ()
            n290 = local write "Blue Error Out"(w488) -> ()
          }
          frame #1 {
            n291 = local write "Initialize Blue Laser"(FALSE ("Initialize")) -> ()
          }
        }
      }
      event "Blue Laser Modluation Mode": Value Change {
        # "Changes the type of modulation for the blue laser"
        n292 = event-data() -> ()  [unwired: 1 in, 5 out]
        n293 = case shown="\"Constant Power\"" "Blue Laser Modluation Mode" {
          tunnel: ["sdmes 1" w522 "sdmes 1" "sdmes 0"] -> w507
          tunnel: ["sames 1" "cp" "sames 0" "sames 1"] -> w506
          frame "Digital + Analog", Default {
          }
          frame "Constant Power" {
            n294 = local read "Blue Laser\nModulation\nPower (mW)"() -> (w525:string)
            n295 = Decimal String To Number(string=w525) -> (number=w521:i32)  [unwired: 2 in, 1 out]
            n296 = Divide(x=w521, y=1000) -> (x/y=w519:dbl)
            n297 = Number To Fractional String(number=w519) -> (F-format string=w520:string)  [unwired: 3 in]
            n298 = Concatenate Strings("p ", w520) -> (w522:string)
          }
          frame "Digital Only" {
          }
          frame "Analog Only" {
          }
        }
        n299 = local read "Delay (ms)"() -> (w516:i32)
        n300 = call "serial write macro.vi"("String"=w507, "Delay (ms)"=w516, "VISA resource name"=w513) -> ("read buffer"=w514:string, "error out"=w515:errorcluster, "VISA resource name out"=w508:refnum<visa-resource-name>)
        n301 = local write "read blue buffer"(w514) -> ()
        n302 = local write "Blue Error Out"(w515) -> ()
        n303 = local read "Delay (ms)"() -> (w511:i32)
        n304 = call "serial write macro.vi"("String"=w506, "Delay (ms)"=w511, "VISA resource name"=w508) -> ("read buffer"=w509:string, "error out"=w510:errorcluster)  [unwired: 1 out]
        n305 = local write "Blue Error Out"(w510) -> ()
        n306 = local write "read blue buffer"(w509) -> ()
      }
      event "Blue Laser\nModulation\nPower (mW)": Value Change {
        n307 = event-data() -> ()  [unwired: 1 in, 5 out]
        n308 = local read "Blue Laser\nModulation\nPower (mW)"() -> (w532:string)
        n309 = local read "Blue Laser Modluation Mode"() -> (w533:string)
        n310 = case shown="\"Constant Power\"" w533 {
          tunnel: w532 -> [w539 w546]
          tunnel: [w538 w545] -> w531
          frame "Constant Power" {
            # "Different command to change constant power instead of modulation power"
            n311 = Decimal String To Number(string=w539) -> (offset past number=w544:i32)  [unwired: 2 in, 1 out]
            n312 = Divide(x=w544, y=1000) -> (x/y=w542:dbl)
            n313 = Number To Fractional String(number=w542) -> (F-format string=w540:string)  [unwired: 3 in]
            n314 = Concatenate Strings("p ", w540) -> (w538:string)
          }
          frame Default {
            n315 = Concatenate Strings("slmp ", w546) -> (w545:string)
          }
        }
        n316 = local read "Delay (ms)"() -> (w536:i32)
        n317 = call "serial write macro.vi"("String"=w531, "Delay (ms)"=w536, "VISA resource name"=w537) -> ("read buffer"=w535:string, "error out"=w534:errorcluster)  [unwired: 1 out]
        n318 = local write "Blue Error Out"(w534) -> ()
        n319 = local write "read blue buffer"(w535) -> ()
      }
      event "Send string\nto Blue Laser": Value Change {
        n320 = event-data() -> ()  [unwired: 1 in, 5 out]
        n321 = flat-sequence {
          tunnel: w548 -> [w553]
          frame #0 {
            n322 = local read "Delay (ms)"() -> (w550:i32)
            n323 = call "serial write macro.vi"("String"="command string", "Delay (ms)"=w550, "VISA resource name"=w553) -> ("read buffer"=w551:string, "error out"=→"Blue Error Out":errorcluster)  [unwired: 1 out]
            "read blue buffer" <- w551
            n324 = String Length(string=w551) -> (length=→"length":i32)
            "command string sent" <- "command string"
          }
          frame #1 {
            n325 = local write "Send string\nto Blue Laser"(FALSE ("Send string")) -> ()
          }
        }
      }
      event "Read Harvard": Value Change {
        n326 = event-data() -> ()  [unwired: 1 in, 5 out]
        n327 = Concatenate Strings("write buffer", "\r") -> (w560:string)
        n328 = VISA Write(VISA resource name=w558, write buffer=w560, error in (no error)=w557) -> (VISA resource name out=w569:refnum<visa-resource-name>, error out=w568:errorcluster)  [unwired: 1 out]
        n329 = stacked-sequence {
          tunnel: [w572] -> w567
          tunnel: w569 -> [w572]
          tunnel: w568 -> [w571]
          tunnel: [w571] -> w562
          frame #0 {
            n330 = Wait (ms)(milliseconds to wait=50) -> ()  [unwired: 1 out]
          }
        }
        n331 = property class="Instr"(reference=w567, error in=w562) -> (reference out=w566:refnum<visa-resource-name>, error out=w564:errorcluster, "Serial Settings:Number of Bytes at Serial Port"=w565:u32)
        "Serial Settings:Number of Bytes at Serial Port" <- w565
        n332 = VISA Read(VISA resource name=w566, byte count=w565, error in (no error)=w564) -> (read buffer=w563:string)  [unwired: 3 out]
        "read buffer" <- w563
        n333 = Fract/Exp String To Number(string=w563) -> ()  [unwired: 5 out]
      }
      event "+z", "-z": Value Change {
        n334 = event-data() -> ()  [unwired: 1 in, 5 out]
        n335 = flat-sequence {
          tunnel: w573 -> [w595]
          tunnel: w574 -> [w575]
          frame #0 {
            n336 = call "Read Stage Position.vi"("error in"=w595, "VISA resource name in"=w575) -> ("Current Position"=w580:cluster{dbl, dbl, dbl}, "error out"=w593:errorcluster, "VISA resource name out"=w594:refnum<visa-resource-name>)  [unwired: 1 out]
            n337 = local read "Saved Stage Positions"() -> (w604:dbl[][])
            n338 = Divide(x="z nudge increment (um)", y=1000.0) -> (x/y=w592:dbl)
            n339 = Boolean To (0,1)(Boolean="+z") -> (0, 1=w584:i16)
            n340 = Boolean To (0,1)(Boolean="-z") -> (0, 1=w585:i16)
            n341 = Array Subset(array=w604, index (row)=1 ("index"), length (row)=1 ("length"), index (col)=1 ("index"), length (col)=3 ("length")) -> (w601:dbl[][])
            n342 = Multiply(x=w584, y=w592) -> (x*y=w588:dbl)
            n343 = Multiply(x=w585, y=w592) -> (x*y=w586:dbl)
            n344 = Unbundle(w580) -> (w578:dbl, w577:dbl, w581:dbl)
            n345 = Negate(x=w586) -> (-x=w587:dbl)
            n346 = Reshape Array(w601, 3 ("dimension size")) -> (w599:dbl[])
            n347 = Add(x=w588, y=w587) -> (x+y=w589:dbl)
            n348 = Array To Cluster(array=w599) -> ()  [unwired: 1 out]
            n349 = Add(x=w589, y=w581) -> (x+y=w579:dbl)
            n350 = Bundle(cluster=w580, w578, w577, w579) -> (w576:cluster{dbl, dbl, dbl})
            n351 = call "Set Stage Position.vi"("Position"=w576, "error in"=w593, "VISA resource name in"=w594) -> ("error out"=w598:errorcluster)  [unwired: 2 out]
            n352 = local write "Stage Moving"(TRUE ("Stage Moving")) -> ()
            n353 = local write "Stage Control Serial Error"(w598) -> ()
          }
          frame #1 {
            n354 = local write "Stage Moving"(FALSE ("Stage Moving")) -> ()
            n355 = call <vilib>:"Beep.vi"() -> ()  [unwired: 3 in, 9 out]
          }
        }
      }
      event "Cal/Data Acq. Spot": Value Change {
        n356 = event-data() -> ()  [unwired: 1 in, 5 out]
        n357 = flat-sequence {
          tunnel: w613 -> [w617]
          tunnel: w614 -> [w618]
          tunnel: [w618] -> w610
          tunnel: [w617] -> w609
          tunnel: w610 -> [w623]
          tunnel: w609 -> [w622]
          tunnel: ["Cal @ (MHz)"] -> w607
          tunnel: [w627] -> w611
          tunnel: w607 -> [w627]
          tunnel: w611 -> [w636]
          tunnel: ["W/ Offset 1"] -> w608
          tunnel: w611 -> [w657]
          tunnel: w608 -> [w655]
          frame #0 {
            n358 = property on="Sample Channel\nFlow" class="Bool (strict)"("Val(Sgnl)"="Daq spot flow on") -> ()  [unwired: 2 in, 2 out]
            n359 = Wait (ms)(milliseconds to wait=u32 250) -> ()  [unwired: 1 out]
          }
          frame #1 {
            n360 = local read "Saved Stage Positions"() -> (w620:dbl[][])
            n361 = property on="Trap Delta (MHz)" class="DigNum (strict)"("Val(Sgnl)"="Cal @ (MHz)") -> ()  [unwired: 2 in, 2 out]
            n362 = local write "Stage Moving"(TRUE ("Stage Moving")) -> ()
            n363 = call "move to saved stage position.vi"("error in"=w622, "Stage VISA resource name in"=w623, "Position"="Cal Stage Position", "Saved Stage Positions"=w620) -> ("error out"=w621:errorcluster)  [unwired: 1 out]
            n364 = local write "Stage Control Serial Error"(w621) -> ()
          }
          frame #2 {
            n365 = local write "Stage Moving"(FALSE ("Stage Moving")) -> ()
            n366 = property on="Sample Channel\nFlow" class="Bool (strict)"("Val(Sgnl)"="Flow ON during cal?") -> ()  [unwired: 2 in, 2 out]
            n367 = call <vilib>:"Beep.vi"() -> ()  [unwired: 3 in, 9 out]
          }
          frame #3 {
            n368 = Wait (ms)(milliseconds to wait=u32 1000) -> ()  [unwired: 1 out]
          }
          frame #4 {
            n369 = property on="Save Calibration" class="Bool (strict)"("Val(Sgnl)"=TRUE ("Value (Signaling)")) -> ()  [unwired: 2 in, 2 out]
          }
          frame #5 {
            n370 = Wait (ms)(milliseconds to wait=u32 2000) -> ()  [unwired: 1 out]
          }
          frame #6 {
            # "Check to see if \nsaving done"
            n371 = while {
              stop <- w632 stop-if-true
              n372 = local read "Saving..."() -> (w633:bool)
              n373 = Wait (ms)(milliseconds to wait=u32 100) -> ()  [unwired: 1 out]
              n374 = Not(x=w633) -> (.not. x?=w632:bool)
            }
          }
          frame #7 {
            n375 = case shown="True" "W/ Offset 1" {
              tunnel: w636 -> [_ w637]
              frame False {
              }
              frame True {
                n376 = stacked-sequence {
                  tunnel: w637 -> [_ _ _ _ _ _ _ w654]
                  frame #0 {
                    n377 = property on="Trap Delta (MHz)" class="DigNum (strict)"("Val(Sgnl)"="Offset 1 Start (MHz)") -> ()  [unwired: 2 in, 2 out]
                    n378 = Replace Array Subset(array=u32[] [0] ("Index Values"), new element="Offset 1 Set", index=0) -> (w638:u32[])
                    n379 = property on="Saved AOD Raster Scan Parameter Sets" class="Arr (strict)"("Index Values"=w638) -> ()  [unwired: 2 in, 2 out]
                  }
                  frame #1 {
                    n380 = Wait (ms)(milliseconds to wait=u32 200) -> ()  [unwired: 1 out]
                  }
                  frame #2 {
                    n381 = property on="Load parameters" class="Bool (strict)"("Val(Sgnl)"=TRUE ("Value (Signaling)")) -> ()  [unwired: 2 in, 2 out]
                  }
                  frame #3 {
                    n382 = Wait (ms)(milliseconds to wait=u32 200) -> ()  [unwired: 1 out]
                  }
                  frame #4 {
                    n383 = property on="Trap Raster Scan" class="Bool (strict)"("Val(Sgnl)"=TRUE ("Value (Signaling)")) -> ()  [unwired: 2 in, 2 out]
                  }
                  frame #5 {
                    n384 = Wait (ms)(milliseconds to wait=u32 2000) -> ()  [unwired: 1 out]
                  }
                  frame #6 {
                    n385 = while {
                      stop <- w651 stop-if-true
                      n386 = local read "Raster Scanning..."() -> (w653:bool)
                      n387 = local read "Saving..."() -> (w649:bool)
                      n388 = Wait (ms)(milliseconds to wait=u32 100) -> ()  [unwired: 1 out]
                      n389 = Not(x=w649) -> (.not. x?=w648:bool)
                      n390 = Not(x=w653) -> (.not. x?=w650:bool)
                      n391 = And(x=w650, y=w648) -> (x .and. y?=w651:bool)
                    }
                  }
                  frame #7 {
                    n392 = property on="Trap Delta (MHz)" class="DigNum (strict)"("Val(Sgnl)"=w654) -> ()  [unwired: 2 in, 2 out]
                  }
                }
              }
            }
          }
          frame #8 {
            n393 = local read "Save ave N"() -> (w656:dbl)
            n394 = case shown="False" "W/ Offset 2" {
              tunnel: w657 -> [_ w664]
              tunnel: w656 -> [_ w663]
              tunnel: w655 -> [w659 _]
              frame False {
                n395 = case shown="False" w659 {
                  frame False {
                    n396 = Multiply(x="Cal read wait (s)", y=u32 1000 ("milliseconds to wait")) -> (x*y=w661:u32)
                    n397 = Wait (ms)(milliseconds to wait=w661) -> ()  [unwired: 1 out]
                  }
                  frame True {
                  }
                }
              }
              frame True {
                n398 = stacked-sequence {